vi "BST106-M10 Weighing Multicontroller Reporter.vi"() -> ()   [LabVIEW 2025]
uses:
  <vilib>/Utility/file.llb/Read Delimited Spreadsheet (string).vi
  Subprogramas/Variable global de carga.vi
  <vilib>/Utility/file.llb/Write Delimited Spreadsheet (string).vi
  <vilib>/Utility/error.llb/Error Cluster From Error Code.vi
  <vilib>/ErrorRing/Error Ring.xnode
  <vilib>/Plasmionique/MB Master/MB_Master_Serial/MB_Master_Serial.lvclass
panel:
  in  "Secret button":bool
  out "ReportXlsxPath":path=path "C:/Temp/Basculas Fabela MultiController/Documentos/Reporte.txt"
  out "CtrlClusterOld":T1(array[cluster])
  out "CtrlNumberOld":i32
  in  "ConfChange":bool caption="Lectura de controladores"
  out "PythonPath":path=path "C:/Temp/Insagro/Documentos/TXTaXLSX.exe"
  out "ReportPath":path=path "C:/Temp/Basculas Fabela MultiController/Documentos/Reporte.txt"
  out "ComNumberPath":path=path "C:/Temp/Basculas Fabela MultiController/Documentos/ComNumber.txt"
  out "ComConfigPath":path=path "C:/Temp/Basculas Fabela MultiController/Documentos/ComConfig.txt"
  out "TxtPath":path=path "C:/Temp/Basculas Fabela MultiController/Documentos/Recetas.txt"
  out "Tabs":enum32{"Home", "Main", "Setup"}(tab)=enum."Setup"
  in  "Controllers Load":T2(array[cluster])=[{"ControlerNum"="Controlador 1", "Recipe"="", "Status"=9868950}] caption="Controladores"
  in  "Carga total":bool
  out "Main Load":enum32{"No load", "Load"}(tab)
  out "Ring 2":u16(ring)
  in  "Read":bool caption="Lectura de controladores"
  out "Loading Text":string
  out "TABLA DE RECETAS":string[][](table)
  in  "SecretAnimationCtrl":i32=1 caption="Selección de animación secreta" min=1
  in  "Array CtrlCluster":T1(array[cluster])=[{"Control#"="Control 1", "Com"=""}]
  in  "CtrlNumber":i32=1 caption="Número de controladores" min=1
  in  "Boton Guardar Cambios":bool
  in  "Settings Nav Button":bool=TRUE
  in  "Recetas Nav Button":bool
  in  "Home Nav Button":bool
  # "Seleccione en cada pantalla la fórmula que desee servir"
  # "Peso Objetivo"
  # "Número de Fórmula"
  # "Peso Servido"
  # "Tolva 1"
  # "Tolva 2"
  # "Tolva 3"
  # "Tolva 4"
  # "Indicador Báscula Sirviendo"
  # "Botón Ajuste Manual"
  # "Indicador Falta Material"
  # "FORMULA SELECCIONADA"
  # "CONFIGURACION DE COMUNICACION"
  # "Seleccione los puertos de comunicación"
  # "Controladores"
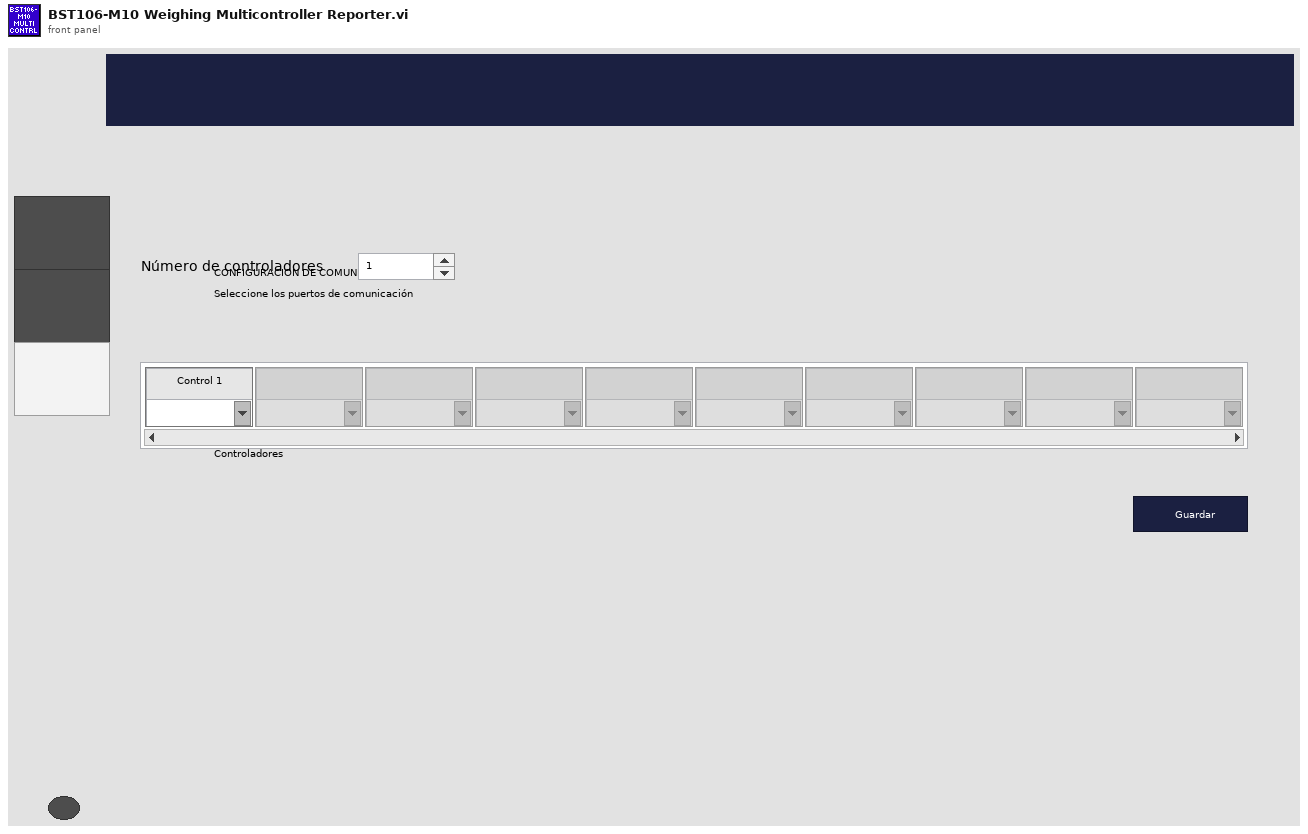
[diagram p1: front panel]
types:
  T1 = cluster{"Control#":string, "Com":refnum<visa-resource-name>}[]
  T2 = cluster{"ControlerNum":string, "Recipe":string, "Status":u32}[]
  T3 = enum8{"Enabled", "Disabled", "Disabled and Grayed Out"}
  T4 = cluster{"Control#":string, "Com":refnum<visa-resource-name>}
  T5 = cluster{"ControlerNum":string, "Recipe":string, "Status":u32}
  T6 = typedef "Control 2.ctl" = refnum<class "MB_Master_Serial.lvclass">[]
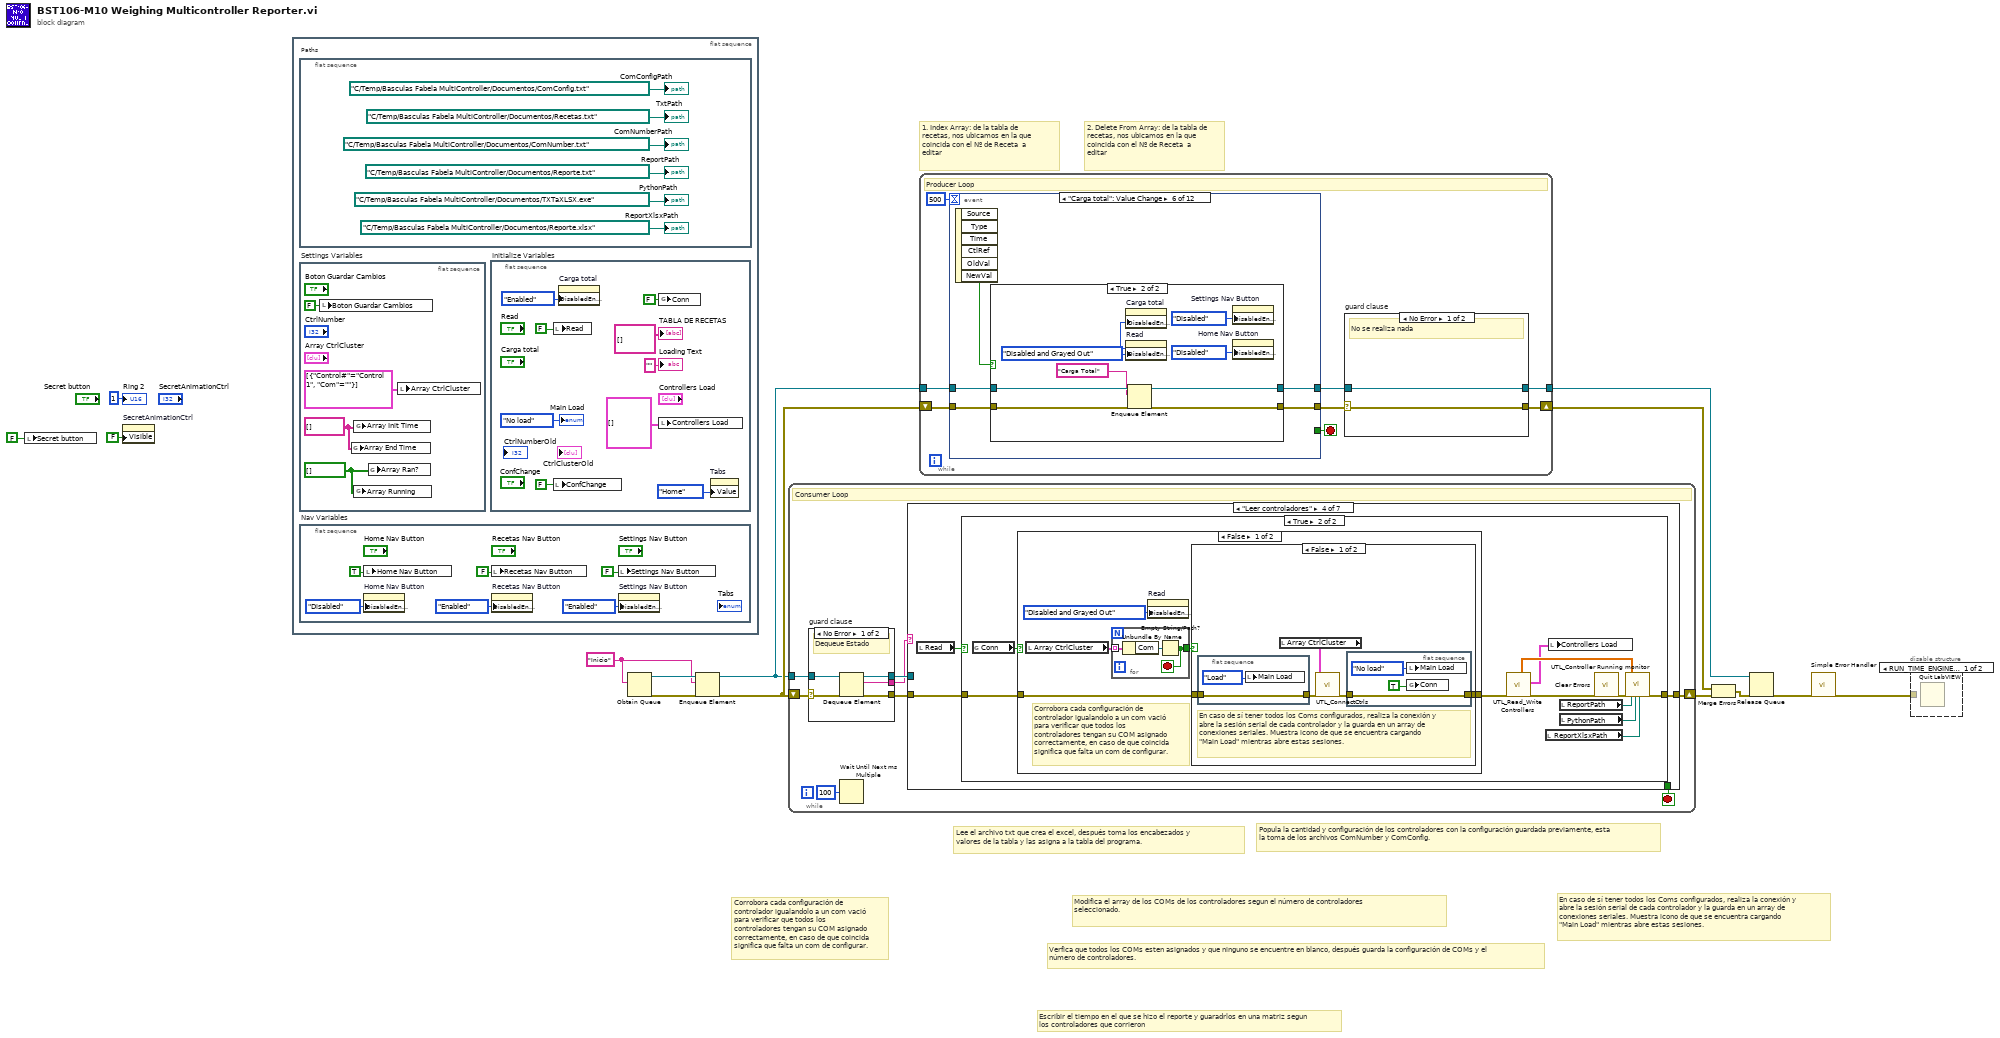
[diagram p0: block diagram]
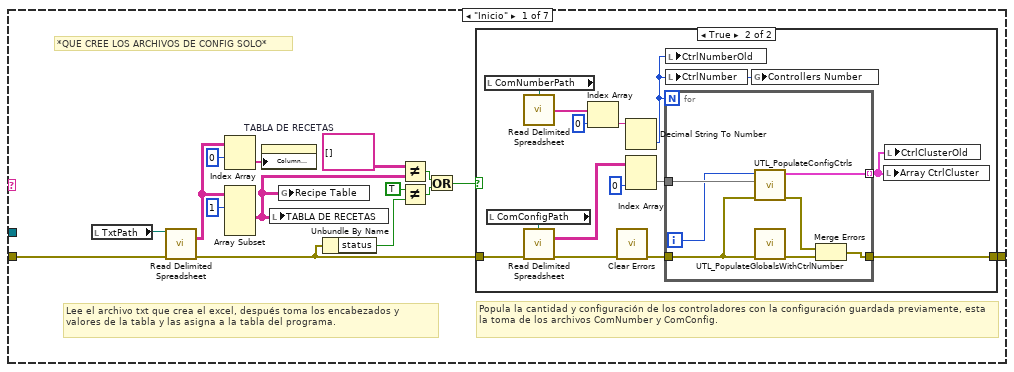
[diagram p2: hidden frame]
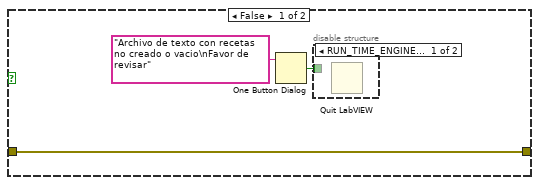
[diagram p3: hidden frame]
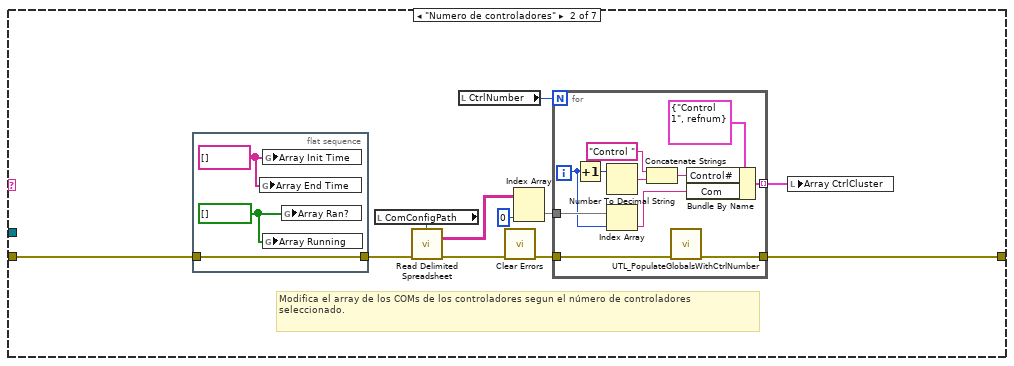
[diagram p5: hidden frame]
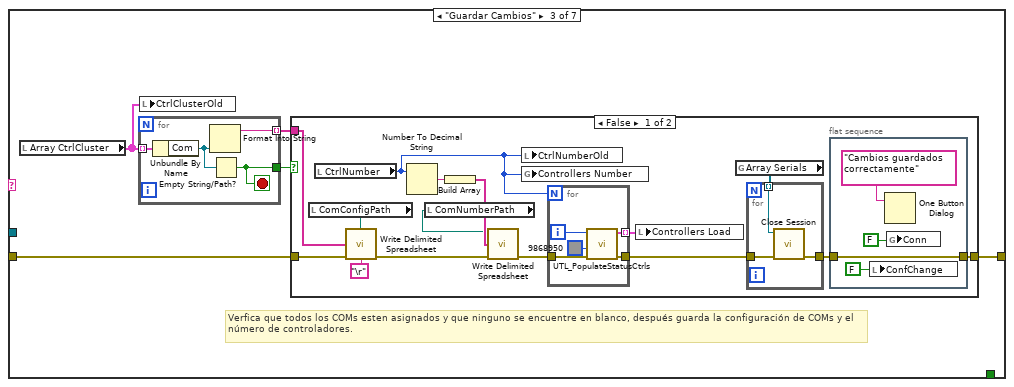
[diagram p6: hidden frame]
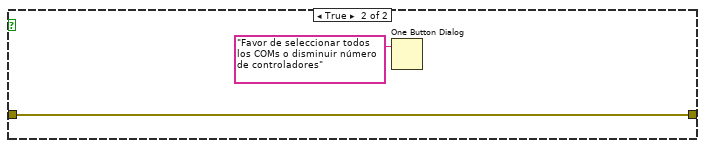
[diagram p7: hidden frame]
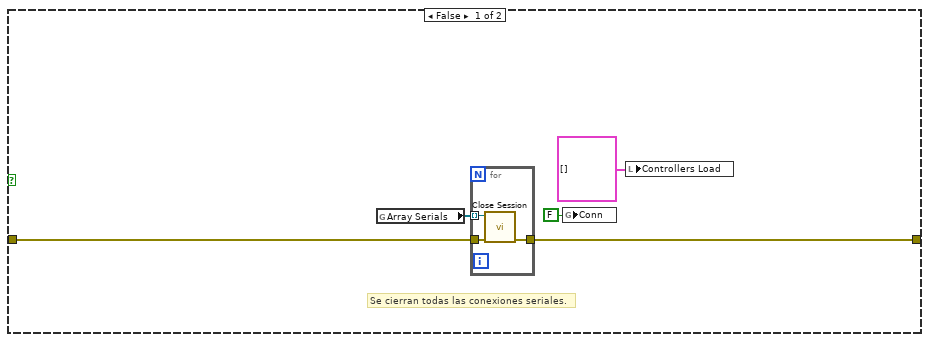
[diagram p8: hidden frame]
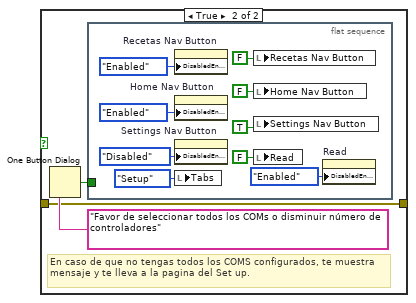
[diagram p9: hidden frame]
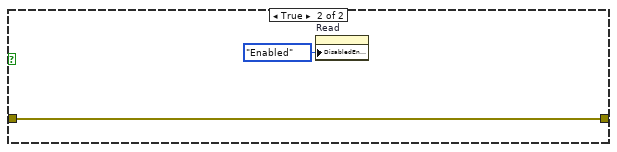
[diagram p10: hidden frame]
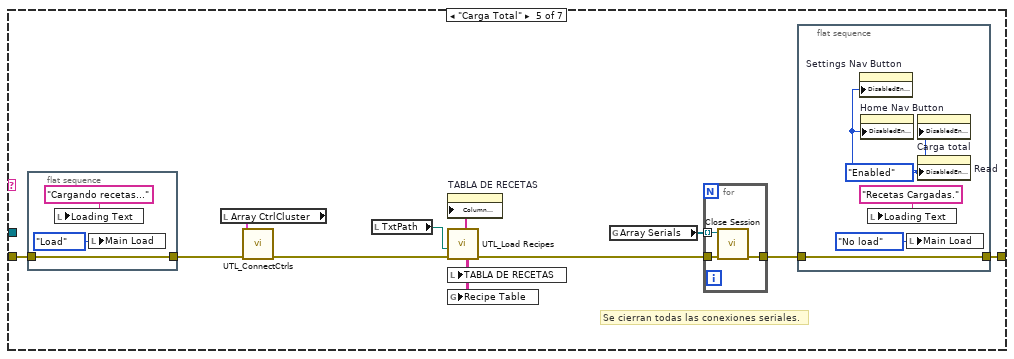
[diagram p11: hidden frame]
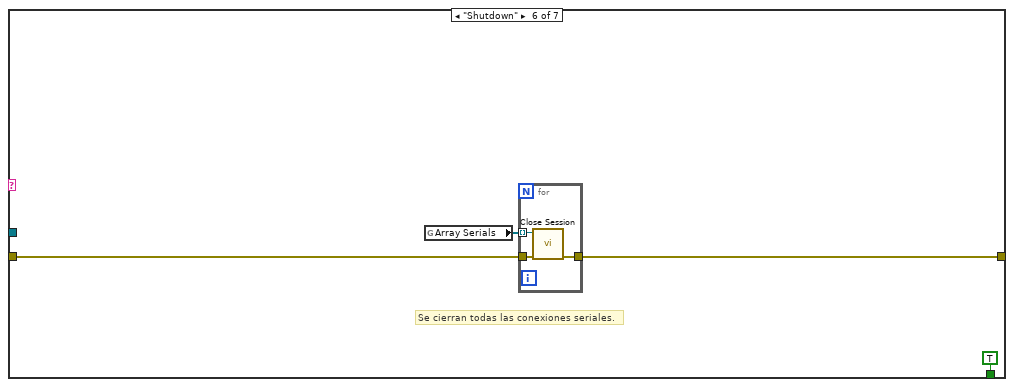
[diagram p12: hidden frame]
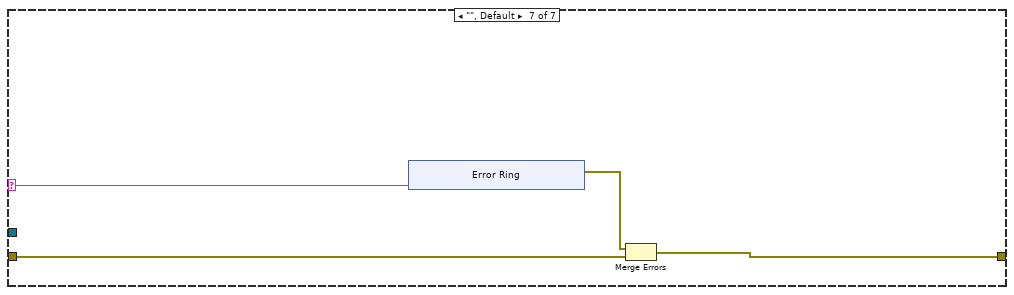
[diagram p13: hidden frame]
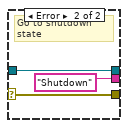
[diagram p14: hidden frame]
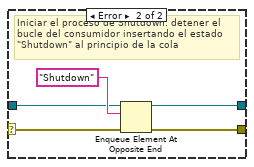
[diagram p15: hidden frame]
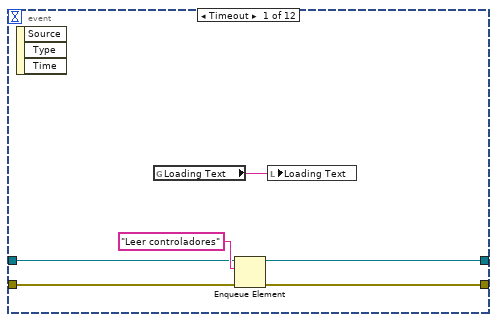
[diagram p16: hidden frame]
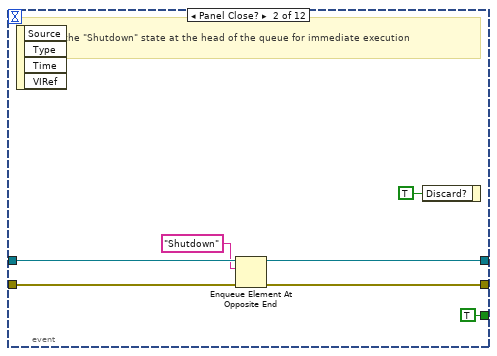
[diagram p17: hidden frame]
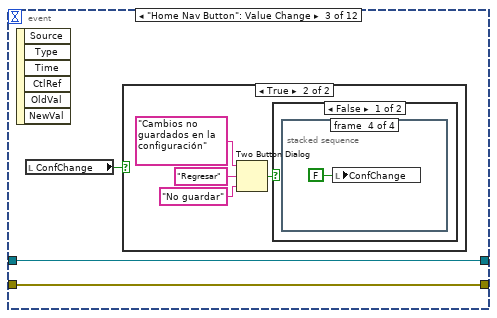
[diagram p18: hidden frame]
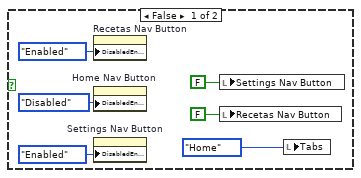
[diagram p19: hidden frame]
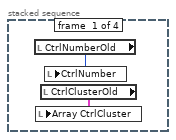
[diagram p20: hidden frame]
diagram:
  w5 = "Inicio"
  # "Escribir el tiempo en el que se hizo el reporte y guaradrlos en una matriz segun los controladores que corrieron"
  # "En caso de sí tener todos los Coms configurados, realiza la conexión y abre la sesión serial de cada controlador y la guarda en un array de conexiones seriales. Muestra icono de que se encuentra cargando \"Main Load\" mientras abre estas sesiones."
  # "Corrobora cada configuración de controlador igualandolo a un com vació para verificar que todos los controladores tengan su COM asignado correctamente, en caso de que coincida significa que falta un com de configurar."
  # "Verfica que todos los COMs esten asignados y que ninguno se encuentre en blanco, después guarda la configuración de COMs y el número de controladores."
  # "Modifica el array de los COMs de los controladores segun el número de controladores seleccionado."
  # "Popula la cantidad y configuración de los controladores con la configuración guardada previamente, esta la toma de los archivos ComNumber y ComConfig."
  # "Lee el archivo txt que crea el excel, después toma los encabezados y valores de la tabla y las asigna a la tabla del programa."
  # "2. Delete From Array: de la tabla de recetas, nos ubicamos en la que coincida con el Nº de Receta  a editar"
  # "1. Index Array: de la tabla de recetas, nos ubicamos en la que coincida con el Nº de Receta  a editar"
  n1 = local write "Secret button"(FALSE ("Secret button")) -> ()
  n2 = property on="SecretAnimationCtrl" class="DigNum (strict)"("Visible"=FALSE) -> ()  [unwired: 2 in, 2 out]
  n3 = flat-sequence {
    frame #0 {
      # "Initialize Variables"
      # "Nav Variables"
      # "Paths"
      # "Settings Variables"
      n4 = flat-sequence {
        frame #0 {
          "TxtPath" <- path "C:/Temp/Basculas Fabela MultiController/Documentos/Recetas.txt" ("name or relative path")
          "ComConfigPath" <- path "C:/Temp/Basculas Fabela MultiController/Documentos/ComConfig.txt" ("name or relative path")
          "ComNumberPath" <- path "C:/Temp/Basculas Fabela MultiController/Documentos/ComNumber.txt" ("name or relative path")
          "ReportPath" <- path "C:/Temp/Basculas Fabela MultiController/Documentos/Reporte.txt" ("name or relative path")
          "PythonPath" <- path "C:/Temp/Basculas Fabela MultiController/Documentos/TXTaXLSX.exe" ("name or relative path")
          "ReportXlsxPath" <- path "C:/Temp/Basculas Fabela MultiController/Documentos/Reporte.xlsx" ("name or relative path")
        }
      }
      n5 = flat-sequence {
        frame #0 {
          w38 = bool[] [] ("Array Ran?")
          w37 = string[] [] ("Array Init Time")
          n6 = local write "Boton Guardar Cambios"(FALSE ("Boton Iniciar programa")) -> ()
          n7 = global write "Variable global de carga.vi" "Array End Time"(w37) -> ()
          n8 = global write "Variable global de carga.vi" "Array Init Time"(w37) -> ()
          n9 = global write "Variable global de carga.vi" "Array Running"(w38) -> ()
          n10 = global write "Variable global de carga.vi" "Array Ran?"(w38) -> ()
          n11 = local write "Array CtrlCluster"(T1 [{"Control#"="Control 1", "Com"=""}] ("Array CtrlCluster")) -> ()
        }
      }
      n12 = flat-sequence {
        frame #0 {
          n13 = local write "Home Nav Button"(TRUE ("Home Nav Button")) -> ()
          n14 = property on="Home Nav Button" class="Bool (strict)"("DisabledEnum"=T3."Disabled" ("Disabled")) -> ()  [unwired: 2 in, 2 out]
          n15 = local write "Recetas Nav Button"(FALSE ("Recetas Nav Button")) -> ()
          n16 = property on="Recetas Nav Button" class="Bool (strict)"("DisabledEnum"=T3."Enabled" ("Disabled")) -> ()  [unwired: 2 in, 2 out]
          n17 = local write "Settings Nav Button"(FALSE ("Settings Nav Button")) -> ()
          n18 = property on="Settings Nav Button" class="Bool (strict)"("DisabledEnum"=T3."Enabled" ("Disabled")) -> ()  [unwired: 2 in, 2 out]
        }
      }
      n19 = flat-sequence {
        frame #0 {
          n20 = local write "Read"(FALSE ("Read")) -> ()
          n21 = local write "ConfChange"(FALSE ("ConfChange")) -> ()
          n22 = property on="Carga total" class="Bool (strict)"("DisabledEnum"=T3."Enabled" ("Disabled")) -> ()  [unwired: 2 in, 2 out]
          n23 = global write "Variable global de carga.vi" "Conn"(FALSE ("Conn")) -> ()
          n24 = local write "Controllers Load"(T2 [] ("Controllers Load")) -> ()
          n25 = property on="Tabs" class="TabCtl (strict)"("Value"=enum32{"Home", "Main", "Setup"}."Home" ("Tab Control")) -> ()  [unwired: 2 in, 2 out]
          "Main Load" <- enum32{"No load", "Load"}."No load" ("Load C1")
          "TABLA DE RECETAS" <- string[][] []
          "Loading Text" <- "" ("Variable de carga")
        }
      }
    }
  }
  n26 = Obtain Queue(element data type=w5) -> (queue out=w14:refnum<queue>, error out=w13:errorcluster)  [unwired: 4 in, 1 out]
  n27 = Enqueue Element(queue=w14, element=w5, error in (no error)=w13) -> (queue out=w8:refnum<queue>, error out=w9:errorcluster)  [unwired: 1 in, 1 out]
  n28 = while {
    shift-right: [w40] -> w11
    shift-left: w9 -> [w47]
    tunnel: w8 -> [w42]
    stop <- w43 stop-if-true
    # "Consumer Loop"
    n29 = case "guard clause" shown="No Error" w47 {
      selector: w47 -> [w247 w250]
      tunnel: [w246 "Shutdown"] -> w41
      tunnel: [w245 w248] -> w46
      tunnel: [w244 w250] -> w45
      tunnel: w42 -> [w243 w248]
      frame No Error {
        # "Dequeue Estado"
        n30 = Dequeue Element(queue=w243, error in (no error)=w247) -> (queue out=w245:refnum<queue>, element=w246:string, error out=w244:errorcluster)  [unwired: 1 in, 1 out]
      }
      frame Error {
        # "Go to shutdown state"
      }
    }
    n31 = Wait Until Next ms Multiple(millisecond multiple=u32 100) -> ()  [unwired: 1 out]
    n32 = case shown="\"Leer controladores\"" w41 {
      selector: w41 -> [_ _ _ _ _ _ w235]
      tunnel: w46 -> [_ _ _ _ _ _ _]
      tunnel: w45 -> [w53 w90 w113 w151 w214 w227 w234]
      tunnel: [_ _ _ _ _ TRUE _] -> w43
      tunnel: [w51 w87 w116 w150 w212 w226 w232] -> w40
      frame "Inicio" {
        # "*QUE CREE LOS ARCHIVOS DE CONFIG SOLO*"
        # "Popula la cantidad y configuración de los controladores con la configuración guardada previamente, esta la toma de los archivos ComNumber y ComConfig."
        # "Lee el archivo txt que crea el excel, después toma los encabezados y valores de la tabla y las asigna a la tabla del programa."
        n33 = local read "TxtPath"() -> (w56:path)
        n34 = call-poly <vilib>:"Read Delimited Spreadsheet.vi"("file path (dialog if empty)"=w56, "error in (no error)"=w53) -> ("all rows"=w61:string[][], "error out"=w52:errorcluster)  [unwired: 8 in, 4 out]
        n35 = Index Array(array=w61, index (row)=0) -> (element=w62:string[])  [unwired: 1 in]
        n36 = Array Subset(array=w61, index (row)=1 ("index")) -> (w50:string[][])  [unwired: 3 in]
        n37 = property on="TABLA DE RECETAS" class="Tbl (strict)"("Column Headers[]"=w62) -> ()  [unwired: 2 in, 2 out]
        n38 = local write "TABLA DE RECETAS"(w50) -> ()
        n39 = global write "Variable global de carga.vi" "Recipe Table"(w50) -> ()
        n40 = Unbundle By Name(w52) -> ("status"=w59:bool)
        n41 = Not Equal?(x=string[][] [], y=w50) -> (x != y?=w58:bool)
        n42 = Not Equal?(x=TRUE, y=w59) -> (x != y?=w60:bool)
        n43 = Or(x=w58, y=w60) -> (x .or. y?=w57:bool)
        n44 = case shown="True" w57 {
          tunnel: w52 -> [w63 w75]
          tunnel: [w63 w68] -> w51
          frame False {
            n45 = One Button Dialog(message="Archivo de texto con recetas no creado o vacio\nFavor de revisar") -> (true=w64:bool)  [unwired: 1 in]
            n46 = disable-structure shown="RUN_TIME_ENGINE==True" {
              disable-tunnel: w64 -> [_ _]
              frame condition #0 {
                n47 = Quit LabVIEW() -> ()  [unwired: 1 in]
              }
              frame condition #1 (active) {
              }
            }
          }
          frame True {
            n48 = local read "ComNumberPath"() -> (w74:path)
            n49 = local read "ComConfigPath"() -> (w76:path)
            n50 = call-poly <vilib>:"Read Delimited Spreadsheet.vi"("file path (dialog if empty)"=w74) -> ("first row"=w73:string[])  [unwired: 9 in, 5 out]
            n51 = call-poly <vilib>:"Read Delimited Spreadsheet.vi"("file path (dialog if empty)"=w76, "error in (no error)"=w75) -> ("all rows"=w79:string[][], "error out"=w77:errorcluster)  [unwired: 8 in, 4 out]
            n52 = Index Array(array=w73, index=0 ("disabled index (col)")) -> (element=w72:string)
            n53 = call <vilib>:"Clear Errors.vi"("error in (no error)"=w77) -> ("error out"=w69:errorcluster)  [unwired: 5 in, 1 out]
            n54 = Decimal String To Number(string=w72) -> (number=w66:i32)  [unwired: 2 in, 1 out]
            n55 = Index Array(array=w79, index (col)=0 ("disabled index (col)")) -> (element=w70:string[])  [unwired: 1 in]
            n56 = for {
              N: w66 -> [_]
              tunnel: w70 -> [w86]
              tunnel: w69 -> [w82]
              tunnel: [w83] -> w68
              tunnel: [w85] -> w67 mode=indexing
              i -> [w81]
              n57 = call "UTL_PopulateConfigCtrls.vi"("error in (no error)"=w82, "ComConfig"=w86, "ComNum"=w81) -> ("error out"=w80:errorcluster, "Array Cluster"=w85:T4)  [unwired: 7 in]
              n58 = call "UTL_PopulateGlobalsWithCtrlNumber.vi"("error in (no error)"=w82) -> ("error out"=w84:errorcluster)  [unwired: 10 in]
              n59 = Merge Errors(w80, w84) -> (w83:errorcluster)
            }
            n60 = local write "CtrlNumberOld"(w66) -> ()
            n61 = local write "CtrlNumber"(w66) -> ()
            n62 = global write "Variable global de carga.vi" "Controllers Number"(w66) -> ()
            n63 = local write "Array CtrlCluster"(w67) -> ()
            n64 = local write "CtrlClusterOld"(w67) -> ()
          }
        }
      }
      frame "Numero de controladores" {
        # "Modifica el array de los COMs de los controladores segun el número de controladores seleccionado."
        n65 = flat-sequence {
          tunnel: w90 -> [w98]
          tunnel: [w98] -> w89
          frame #0 {
            w100 = bool[] [] ("Array Ran?")
            w99 = string[] [] ("Array Init Time")
            n66 = global write "Variable global de carga.vi" "Array End Time"(w99) -> ()
            n67 = global write "Variable global de carga.vi" "Array Init Time"(w99) -> ()
            n68 = global write "Variable global de carga.vi" "Array Running"(w100) -> ()
            n69 = global write "Variable global de carga.vi" "Array Ran?"(w100) -> ()
          }
        }
        n70 = local read "ComConfigPath"() -> (w95:path)
        n71 = call-poly <vilib>:"Read Delimited Spreadsheet.vi"("file path (dialog if empty)"=w95, "error in (no error)"=w89) -> ("all rows"=w97:string[][], "error out"=w96:errorcluster)  [unwired: 8 in, 4 out]
        n72 = local read "CtrlNumber"() -> (w91:i32)
        n73 = call <vilib>:"Clear Errors.vi"("error in (no error)"=w96) -> ("error out"=w88:errorcluster)  [unwired: 5 in, 1 out]
        n74 = Index Array(array=w97, index (col)=0 ("disabled index (col)")) -> (element=w94:string[])  [unwired: 1 in]
        n75 = for {
          N: w91 -> [_]
          tunnel: w94 -> [w105]
          tunnel: [w106] -> w93 mode=indexing
          tunnel: w88 -> [w102]
          tunnel: [w101] -> w87
          i -> [w104]
          n76 = Increment(x=w104) -> (x+1=w107:i32)
          n77 = Number To Decimal String(number=w107) -> (decimal integer string=w111:string)  [unwired: 1 in]
          n78 = Index Array(array=w105, index=w104) -> (element=w103:string)
          n79 = Concatenate Strings("Control " ("Control#"), w111) -> (w110:string)
          n80 = call "UTL_PopulateGlobalsWithCtrlNumber.vi"("error in (no error)"=w102) -> ("error out"=w101:errorcluster)  [unwired: 10 in]
          n81 = Bundle By Name(cluster=T4 {"Control#"="Control 1", "Com"=""} ("CtrlClust"), "Control#"=w110, "Com"=w103) -> (w106:T4)
        }
        n82 = local write "Array CtrlCluster"(w93) -> ()
      }
      frame "Guardar Cambios" {
        # "Verfica que todos los COMs esten asignados y que ninguno se encuentre en blanco, después guarda la configuración de COMs y el número de controladores."
        n83 = local read "Array CtrlCluster"() -> (w112:T1)
        n84 = for {
          tunnel: [w146] -> w114
          tunnel: [w149] -> w115 mode=indexing
          tunnel: w112 -> [w148] mode=indexing
          stop <- w146 stop-if-true
          n85 = Unbundle By Name(w148) -> ("Com"=w147:refnum<visa-resource-name>)
          n86 = Format Into String(w147) -> (resulting string=w149:string)  [unwired: 3 in, 1 out]
          n87 = Empty String/Path?(string/path=w147) -> (empty?=w146:bool)
        }
        n88 = local write "CtrlClusterOld"(w112) -> ()
        n89 = case shown="False" w114 {
          tunnel: w115 -> [w130 _]
          tunnel: [w126 w144] -> w116
          tunnel: w113 -> [w129 w144]
          frame False {
            n90 = local read "ComConfigPath"() -> (w128:path)
            n91 = local read "CtrlNumber"() -> (w117:i32)
            n92 = call-poly <vilib>:"Write Delimited Spreadsheet.vi"("file path (dialog if empty)"=w128, "1D data"=w130, "error in (no error)"=w129, "delimiter (\\t)"="\r") -> ("error out"=w122:errorcluster)  [unwired: 10 in, 1 out]
            n93 = Number To Decimal String(number=w117) -> (decimal integer string=w124:string)  [unwired: 1 in]
            n94 = local read "ComNumberPath"() -> (w121:path)
            n95 = Build Array(w124) -> (w123:string[])
            n96 = call-poly <vilib>:"Write Delimited Spreadsheet.vi"("file path (dialog if empty)"=w121, "1D data"=w123, "error in (no error)"=w122) -> ("error out"=w120:errorcluster)  [unwired: 11 in, 1 out]
            n97 = local write "CtrlNumberOld"(w117) -> ()
            n98 = global write "Variable global de carga.vi" "Controllers Number"(w117) -> ()
            n99 = for {
              N: w117 -> [_]
              tunnel: w120 -> [w136]
              tunnel: [w135] -> w119
              tunnel: [w132] -> w118 mode=indexing
              i -> [w133]
              n100 = call "UTL_PopulateStatusCtrls.vi"("error in (no error)"=w136, "Status"=u32 9868950, "ComNum"=w133) -> ("error out"=w135:errorcluster, "output cluster"=w132:T5)  [unwired: 7 in]
            }
            n101 = local write "Controllers Load"(w118) -> ()
            n102 = global read "Variable global de carga.vi" "Array Serials"() -> (w125:T6)
            n103 = for {
              tunnel: [w143] -> w127
              tunnel: w119 -> [w142]
              tunnel: w125 -> [w141] mode=indexing
              n104 = call-dynamic "Close Session.vi"("error in (no error)"=w142, "MB_Serial session"=w141) -> ("error out"=w143:errorcluster)  [unwired: 9 in]
            }
            n105 = flat-sequence {
              tunnel: w127 -> [w140]
              tunnel: [w140] -> w126
              frame #0 {
                n106 = local write "ConfChange"(FALSE ("ConfChange")) -> ()
                n107 = One Button Dialog(message="Cambios guardados correctamente") -> ()  [unwired: 1 in, 1 out]
                n108 = global write "Variable global de carga.vi" "Conn"(FALSE ("Conn")) -> ()
              }
            }
          }
          frame True {
            n109 = One Button Dialog(message="Favor de seleccionar todos los COMs o disminuir número de controladores") -> ()  [unwired: 1 in, 1 out]
          }
        }
      }
      frame "Leer controladores" {
        n110 = local read "Read"() -> (w152:bool)
        n111 = case shown="True" w152 {
          tunnel: [w155 w171] -> w150
          tunnel: w151 -> [w156 w165]
          frame False {
            # "Se cierran todas las conexiones seriales."
            n112 = global read "Variable global de carga.vi" "Array Serials"() -> (w157:T6)
            n113 = for {
              tunnel: [w160] -> w155
              tunnel: w156 -> [w159]
              tunnel: w157 -> [w158] mode=indexing
              n114 = call-dynamic "Close Session.vi"("error in (no error)"=w159, "MB_Serial session"=w158) -> ("error out"=w160:errorcluster)  [unwired: 9 in]
            }
            n115 = global write "Variable global de carga.vi" "Conn"(FALSE ("Conn")) -> ()
            n116 = local write "Controllers Load"(T2 [] ("Controllers Load")) -> ()
          }
          frame True {
            n117 = global read "Variable global de carga.vi" "Conn"() -> (w167:bool)
            n118 = case shown="False" w167 {
              tunnel: [w176 w203] -> w166
              tunnel: w165 -> [w173 w203]
              frame False {
                # "Corrobora cada configuración de controlador igualandolo a un com vació para verificar que todos los controladores tengan su COM asignado correctamente, en caso de que coincida significa que falta un com de configurar."
                n119 = local read "Array CtrlCluster"() -> (w174:T1)
                n120 = for {
                  tunnel: [w177] -> w175
                  tunnel: w174 -> [w179] mode=indexing
                  stop <- w177 stop-if-true
                  n121 = Unbundle By Name(w179) -> ("Com"=w178:refnum<visa-resource-name>)
                  n122 = Empty String/Path?(string/path=w178) -> (empty?=w177:bool)
                }
                n123 = property on="Read" class="Bool (strict)"("DisabledEnum"=T3."Disabled and Grayed Out" ("Disabled")) -> ()  [unwired: 2 in, 2 out]
                n124 = case shown="False" w175 {
                  tunnel: [w184 w190] -> w176
                  tunnel: w173 -> [w180 w190]
                  frame False {
                    # "En caso de sí tener todos los Coms configurados, realiza la conexión y abre la sesión serial de cada controlador y la guarda en un array de conexiones seriales. Muestra icono de que se encuentra cargando \"Main Load\" mientras abre estas sesiones."
                    n125 = flat-sequence {
                      tunnel: [w188] -> w181
                      tunnel: w180 -> [w188]
                      frame #0 {
                        n126 = local write "Main Load"(enum32{"No load", "Load"}."Load" ("Load C1")) -> ()
                      }
                    }
                    n127 = local read "Array CtrlCluster"() -> (w182:T1)
                    n128 = call "UTL_ConnectCtrls.vi"("error in (no error)"=w181, "Array CtrlCluster"=w182) -> ("error out"=w183:errorcluster)  [unwired: 9 in]
                    n129 = flat-sequence {
                      tunnel: w183 -> [w186]
                      tunnel: [w186] -> w184
                      frame #0 {
                        n130 = local write "Main Load"(enum32{"No load", "Load"}."No load" ("Load C1")) -> ()
                        n131 = global write "Variable global de carga.vi" "Conn"(TRUE ("Conn")) -> ()
                      }
                    }
                  }
                  frame True {
                    # "En caso de que no tengas todos los COMS configurados, te muestra mensaje y te lleva a la pagina del Set up."
                    n132 = One Button Dialog(message="Favor de seleccionar todos los COMs o disminuir número de controladores") -> (true=w191:bool)  [unwired: 1 in]
                    n133 = flat-sequence {
                      tunnel: w191 -> [_]
                      frame #0 {
                        n134 = property on="Recetas Nav Button" class="Bool (strict)"("DisabledEnum"=T3."Enabled" ("Disabled")) -> ()  [unwired: 2 in, 2 out]
                        n135 = property on="Home Nav Button" class="Bool (strict)"("DisabledEnum"=T3."Enabled" ("Disabled")) -> ()  [unwired: 2 in, 2 out]
                        n136 = property on="Settings Nav Button" class="Bool (strict)"("DisabledEnum"=T3."Disabled" ("Disabled")) -> ()  [unwired: 2 in, 2 out]
                        n137 = local write "Tabs"(enum32{"Home", "Main", "Setup"}."Setup" ("Pagina programa")) -> ()
                        n138 = local write "Recetas Nav Button"(FALSE ("Recetas Nav Button")) -> ()
                        n139 = local write "Home Nav Button"(FALSE ("Settings Nav Button")) -> ()
                        n140 = local write "Settings Nav Button"(TRUE ("Settings Nav Button")) -> ()
                        n141 = local write "Read"(FALSE ("Read")) -> ()
                        n142 = property on="Read" class="Bool (strict)"("DisabledEnum"=T3."Enabled" ("Disabled")) -> ()  [unwired: 2 in, 2 out]
                      }
                    }
                  }
                }
              }
              frame True {
                n143 = property on="Read" class="Bool (strict)"("DisabledEnum"=T3."Enabled" ("Disabled")) -> ()  [unwired: 2 in, 2 out]
              }
            }
            n144 = call "UTL_Read_Write Controllers.vi"("error in"=w166) -> ("error out"=w170:errorcluster, "StatusCtrl"=w168:T2, "Results"=w169:dbl[][][])  [unwired: 8 in]
            n145 = local read "ReportXlsxPath"() -> (w161:path)
            n146 = local write "Controllers Load"(w168) -> ()
            n147 = local read "ReportPath"() -> (w163:path)
            n148 = local read "PythonPath"() -> (w162:path)
            n149 = call <vilib>:"Clear Errors.vi"("error in (no error)"=w170) -> ("error out"=w164:errorcluster)  [unwired: 5 in, 1 out]
            n150 = call "UTL_Controller Running monitor.vi"("Error In"=w164, "Data"=w169, "ReportPath"=w163, "PyPath"=w162, "ReportXlsxPath"=w161) -> ("Error Out"=w171:errorcluster)  [unwired: 14 in]
          }
        }
      }
      frame "Carga Total" {
        # "Se cierran todas las conexiones seriales."
        n151 = flat-sequence {
          tunnel: w214 -> [w223]
          tunnel: [w223] -> w208
          frame #0 {
            n152 = local write "Loading Text"("Cargando recetas..." ("Carga texto")) -> ()
            n153 = local write "Main Load"(enum32{"No load", "Load"}."Load" ("Load C1")) -> ()
          }
        }
        n154 = local read "Array CtrlCluster"() -> (w209:T1)
        n155 = call "UTL_ConnectCtrls.vi"("error in (no error)"=w208, "Array CtrlCluster"=w209) -> ("error out"=w207:errorcluster)  [unwired: 9 in]
        n156 = local read "TxtPath"() -> (w213:path)
        n157 = call "UTL_Load Recipes.vi"("Error in"=w207, "Txt Path"=w213) -> ("Error out"=w205:errorcluster, "Headers"=w210:string[], "Sorted 2D table array"=w211:string[][])  [unwired: 7 in]
        n158 = property on="TABLA DE RECETAS" class="Tbl (strict)"("Column Headers[]"=w210) -> ()  [unwired: 2 in, 2 out]
        n159 = local write "TABLA DE RECETAS"(w211) -> ()
        n160 = global write "Variable global de carga.vi" "Recipe Table"(w211) -> ()
        n161 = global read "Variable global de carga.vi" "Array Serials"() -> (w206:T6)
        n162 = for {
          tunnel: [w217] -> w204
          tunnel: w205 -> [w216]
          tunnel: w206 -> [w215] mode=indexing
          n163 = call-dynamic "Close Session.vi"("error in (no error)"=w216, "MB_Serial session"=w215) -> ("error out"=w217:errorcluster)  [unwired: 9 in]
        }
        n164 = flat-sequence {
          tunnel: w204 -> [w220]
          tunnel: [w220] -> w212
          frame #0 {
            w218 = T3."Enabled" ("Disabled")
            n165 = property on="Settings Nav Button" class="Bool (strict)"("DisabledEnum"=w218) -> ()  [unwired: 2 in, 2 out]
            n166 = property on="Home Nav Button" class="Bool (strict)"("DisabledEnum"=w218) -> ()  [unwired: 2 in, 2 out]
            n167 = local write "Loading Text"("Recetas Cargadas." ("Carga texto")) -> ()
            n168 = local write "Main Load"(enum32{"No load", "Load"}."No load" ("Load C1")) -> ()
            n169 = property on="Carga total" class="Bool (strict)"("DisabledEnum"=w218) -> ()  [unwired: 2 in, 2 out]
            n170 = property on="Read" class="Bool (strict)"("DisabledEnum"=w218) -> ()  [unwired: 2 in, 2 out]
          }
        }
      }
      frame "Shutdown" {
        # "Se cierran todas las conexiones seriales."
        # "Stop the Consumer Loop, and signal the Producer Loop to also stop by activating the front-panel \"Stop\" button; use the \"signaling\" version to trigger the event structure"
        n171 = global read "Variable global de carga.vi" "Array Serials"() -> (w225:T6)
        n172 = for {
          tunnel: [w231] -> w226
          tunnel: w227 -> [w230]
          tunnel: w225 -> [w229] mode=indexing
          n173 = call-dynamic "Close Session.vi"("error in (no error)"=w230, "MB_Serial session"=w229) -> ("error out"=w231:errorcluster)  [unwired: 9 in]
        }
      }
      frame "", Default {
        # "Handle unknown states"
        n174 = xnode "Error Ring"("parameter 0"=w235) -> ("error out"=w233:errorcluster)
        n175 = Merge Errors(w233, w234) -> (w232:errorcluster)
      }
    }
  }
  n176 = while {
    shift-right: [w253] -> w7
    shift-left: w9 -> [w257]
    tunnel: w8 -> [w256]
    tunnel: [w254] -> w6
    stop <- w252 stop-if-true
    # "Producer Loop"
    n177 = event shown="[5] \"Carga total\": Value Change" {
      selector: _ -> [_ _ _ _ _ _ _ _ _ _ _ _]
      dyn-events: _ -> [_ _ _ _ _ _ _ _ _ _ _ _]
      timeout: 500 -> [_ _ _ _ _ _ _ _ _ _ _ _]
      tunnel: [w268 w275 w280 w306 w335 w339 w356 w364 w371 _ _ w387] -> w258
      tunnel: w257 -> [w269 w276 w280 w306 w335 w340 w357 w364 w371 _ _ w388]
      tunnel: w256 -> [w266 w278 w281 w305 w334 w341 w359 w365 w370 _ _ w389]
      tunnel: [_ TRUE _ _ _ _ _ _ _ _ _ _] -> w252
      tunnel: [w267 w273 w281 w305 w334 w338 w355 w365 w370 _ _ w386] -> w255
      event Timeout {
        n178 = event-data() -> ()  [unwired: 1 in, 3 out]
        n179 = global read "Variable global de carga.vi" "Loading Text"() -> (w271:string)
        n180 = Enqueue Element(queue=w266, element="Leer controladores", error in (no error)=w269) -> (queue out=w267:refnum<queue>, error out=w268:errorcluster)  [unwired: 1 in, 1 out]
        n181 = local write "Loading Text"(w271) -> ()
      }
      event Panel Close? {
        # "Enqueue the \"Shutdown\" state at the head of the queue for immediate execution"
        n182 = event-data() -> ()  [unwired: 1 in, 4 out]
        n183 = Enqueue Element At Opposite End(queue=w278, element="Shutdown", error in (no error)=w276) -> (queue out=w273:refnum<queue>, error out=w275:errorcluster)  [unwired: 1 in, 1 out]
        n184 = event-data("Discard?"=TRUE) -> ()  [unwired: 1 in, 1 out]
      }
      event "Home Nav Button": Value Change {
        n185 = event-data() -> ()  [unwired: 1 in, 6 out]
        n186 = local read "ConfChange"() -> (w279:bool)
        n187 = case shown="True" w279 {
          frame False {
            n188 = property on="Recetas Nav Button" class="Bool (strict)"("DisabledEnum"=T3."Enabled" ("Disabled")) -> ()  [unwired: 2 in, 2 out]
            n189 = property on="Home Nav Button" class="Bool (strict)"("DisabledEnum"=T3."Disabled" ("Disabled")) -> ()  [unwired: 2 in, 2 out]
            n190 = property on="Settings Nav Button" class="Bool (strict)"("DisabledEnum"=T3."Enabled" ("Disabled")) -> ()  [unwired: 2 in, 2 out]
            n191 = local write "Settings Nav Button"(FALSE ("Settings Nav Button")) -> ()
            n192 = local write "Recetas Nav Button"(FALSE ("Recetas Nav Button")) -> ()
            n193 = local write "Tabs"(enum32{"Home", "Main", "Setup"}."Home" ("Pagina programa")) -> ()
          }
          frame True {
            n194 = Two Button Dialog(message="Cambios no guardados en la configuración", 1:"No guardar" ("F button name (\"Cancel\")"), 2:"Regresar" ("T button name (\"OK\")")) -> (T button?=w288:bool)
            n195 = case shown="False" w288 {
              frame False {
                n196 = stacked-sequence {
                  frame #0 {
                    n197 = local read "CtrlNumberOld"() -> (w292:i32)
                    n198 = local read "CtrlClusterOld"() -> (w293:T1)
                    n199 = local write "Array CtrlCluster"(w293) -> ()
                    n200 = local write "CtrlNumber"(w292) -> ()
                  }
                  frame #1 {
                    w295 = T3."Enabled" ("Disabled")
                    n201 = property on="Settings Nav Button" class="Bool (strict)"("DisabledEnum"=w295) -> ()  [unwired: 2 in, 2 out]
                    n202 = property on="Recetas Nav Button" class="Bool (strict)"("DisabledEnum"=w295) -> ()  [unwired: 2 in, 2 out]
                    n203 = property on="Home Nav Button" class="Bool (strict)"("DisabledEnum"=T3."Disabled" ("Disabled")) -> ()  [unwired: 2 in, 2 out]
                  }
                  frame #2 {
                    n204 = local write "Settings Nav Button"(FALSE ("Settings Nav Button")) -> ()
                    n205 = local write "Recetas Nav Button"(FALSE ("Recetas Nav Button")) -> ()
                    n206 = local write "Tabs"(enum32{"Home", "Main", "Setup"}."Home" ("Pagina programa")) -> ()
                  }
                  frame #3 {
                    n207 = local write "ConfChange"(FALSE ("ConfChange")) -> ()
                  }
                }
              }
              frame True {
                n208 = local write "Recetas Nav Button"(FALSE ("Recetas Nav Button")) -> ()
                n209 = local write "Home Nav Button"(FALSE ("Settings Nav Button")) -> ()
                n210 = local write "Settings Nav Button"(TRUE ("Settings Nav Button")) -> ()
                n211 = local write "Tabs"(enum32{"Home", "Main", "Setup"}."Setup" ("Pagina programa")) -> ()
              }
            }
          }
        }
      }
      event "Recetas Nav Button": Value Change {
        n212 = event-data() -> ()  [unwired: 1 in, 6 out]
        n213 = local read "ConfChange"() -> (w304:bool)
        n214 = case shown="True" w304 {
          frame False {
            n215 = property on="Recetas Nav Button" class="Bool (strict)"("DisabledEnum"=T3."Disabled" ("Disabled")) -> ()  [unwired: 2 in, 2 out]
            n216 = property on="Home Nav Button" class="Bool (strict)"("DisabledEnum"=T3."Enabled" ("Disabled")) -> ()  [unwired: 2 in, 2 out]
            n217 = property on="Settings Nav Button" class="Bool (strict)"("DisabledEnum"=T3."Enabled" ("Disabled")) -> ()  [unwired: 2 in, 2 out]
            n218 = local write "Home Nav Button"(FALSE ("Recetas Nav Button")) -> ()
            n219 = local write "Settings Nav Button"(FALSE ("Settings Nav Button")) -> ()
            n220 = local write "Tabs"(enum32{"Home", "Main", "Setup"}."Main" ("Pagina programa")) -> ()
          }
          frame True {
            n221 = Two Button Dialog(message="Cambios no guardados en la configuración", 1:"No guardar" ("F button name (\"Cancel\")"), 2:"Regresar" ("T button name (\"OK\")")) -> (T button?=w316:bool)
            n222 = case shown="False" w316 {
              frame False {
                n223 = stacked-sequence {
                  frame #0 {
                    n224 = local read "CtrlNumberOld"() -> (w317:i32)
                    n225 = local read "CtrlClusterOld"() -> (w318:T1)
                    n226 = local write "Array CtrlCluster"(w318) -> ()
                    n227 = local write "CtrlNumber"(w317) -> ()
                  }
                  frame #1 {
                    w320 = T3."Enabled" ("Disabled")
                    n228 = property on="Recetas Nav Button" class="Bool (strict)"("DisabledEnum"=T3."Disabled" ("Disabled")) -> ()  [unwired: 2 in, 2 out]
                    n229 = property on="Home Nav Button" class="Bool (strict)"("DisabledEnum"=w320) -> ()  [unwired: 2 in, 2 out]
                    n230 = property on="Settings Nav Button" class="Bool (strict)"("DisabledEnum"=w320) -> ()  [unwired: 2 in, 2 out]
                  }
                  frame #2 {
                    n231 = local write "Home Nav Button"(FALSE ("Recetas Nav Button")) -> ()
                    n232 = local write "Settings Nav Button"(FALSE ("Settings Nav Button")) -> ()
                    n233 = local write "Tabs"(enum32{"Home", "Main", "Setup"}."Main" ("Pagina programa")) -> ()
                  }
                  frame #3 {
                    n234 = local write "ConfChange"(FALSE ("ConfChange")) -> ()
                  }
                }
              }
              frame True {
                n235 = local write "Recetas Nav Button"(FALSE ("Recetas Nav Button")) -> ()
                n236 = local write "Home Nav Button"(FALSE ("Settings Nav Button")) -> ()
                n237 = local write "Settings Nav Button"(TRUE ("Settings Nav Button")) -> ()
                n238 = local write "Tabs"(enum32{"Home", "Main", "Setup"}."Setup" ("Pagina programa")) -> ()
              }
            }
          }
        }
      }
      event "Settings Nav Button": Value Change {
        n239 = event-data() -> ()  [unwired: 1 in, 6 out]
        n240 = property on="Recetas Nav Button" class="Bool (strict)"("DisabledEnum"=T3."Enabled" ("Disabled")) -> ()  [unwired: 2 in, 2 out]
        n241 = property on="Home Nav Button" class="Bool (strict)"("DisabledEnum"=T3."Enabled" ("Disabled")) -> ()  [unwired: 2 in, 2 out]
        n242 = property on="Settings Nav Button" class="Bool (strict)"("DisabledEnum"=T3."Disabled" ("Disabled")) -> ()  [unwired: 2 in, 2 out]
        n243 = local write "Home Nav Button"(FALSE ("Recetas Nav Button")) -> ()
        n244 = local write "Recetas Nav Button"(FALSE ("Recetas Nav Button")) -> ()
        n245 = local write "Tabs"(enum32{"Home", "Main", "Setup"}."Setup" ("Pagina programa")) -> ()
      }
      event "Carga total": Value Change {
        n246 = event-data() -> ("NewVal"=w337:bool)  [unwired: 1 in, 5 out]
        n247 = case shown="True" w337 {
          tunnel: w341 -> [w343 w351]
          tunnel: w340 -> [w342 w349]
          tunnel: [w342 w348] -> w339
          tunnel: [w343 w347] -> w338
          frame False {
          }
          frame True {
            w346 = T3."Disabled and Grayed Out" ("Disabled")
            n248 = property on="Carga total" class="Bool (strict)"("DisabledEnum"=w346) -> ()  [unwired: 2 in, 2 out]
            n249 = property on="Read" class="Bool (strict)"("DisabledEnum"=w346) -> ()  [unwired: 2 in, 2 out]
            n250 = Enqueue Element(queue=w351, element="Carga Total", error in (no error)=w349) -> (queue out=w347:refnum<queue>, error out=w348:errorcluster)  [unwired: 1 in, 1 out]
            n251 = property on="Settings Nav Button" class="Bool (strict)"("DisabledEnum"=T3."Disabled" ("Disabled")) -> ()  [unwired: 2 in, 2 out]
            n252 = property on="Home Nav Button" class="Bool (strict)"("DisabledEnum"=T3."Disabled" ("Disabled")) -> ()  [unwired: 2 in, 2 out]
          }
        }
      }
      event "CtrlNumber": Value Change {
        n253 = event-data() -> ()  [unwired: 1 in, 6 out]
        n254 = local read "CtrlNumberOld"() -> (w353:i32)
        n255 = local read "CtrlNumber"() -> (w352:i32)
        n256 = Not Equal?(x=w353, y=w352) -> (x != y?=w354:bool)
        n257 = case shown="False" w354 {
          frame False {
            n258 = local write "ConfChange"(FALSE ("ConfChange")) -> ()
          }
          frame True {
            n259 = local write "ConfChange"(TRUE ("ConfChange")) -> ()
          }
        }
        n260 = Enqueue Element(queue=w359, element="Numero de controladores", error in (no error)=w357) -> (queue out=w355:refnum<queue>, error out=w356:errorcluster)  [unwired: 1 in, 1 out]
      }
      event "Array CtrlCluster": Value Change {
        n261 = event-data() -> ()  [unwired: 1 in, 6 out]
        n262 = local read "Array CtrlCluster"() -> (w362:T1)
        n263 = local read "CtrlClusterOld"() -> (w363:T1)
        n264 = Not Equal?(x=w363, y=w362) -> (x != y?=w366:bool)
        n265 = case shown="True" w366 {
          frame False {
            n266 = local write "ConfChange"(FALSE ("ConfChange")) -> ()
          }
          frame True {
            n267 = local write "ConfChange"(TRUE ("ConfChange")) -> ()
          }
        }
      }
      event "Read": Value Change {
        n268 = event-data() -> ("NewVal"=w369:bool)  [unwired: 1 in, 5 out]
        n269 = case shown="True" w369 {
          frame False {
            n270 = global write "Variable global de carga.vi" "Conn"(FALSE ("Conn")) -> ()
            n271 = local write "Controllers Load"(T2 [] ("Controllers Load")) -> ()
            n272 = property on="Carga total" class="Bool (strict)"("DisabledEnum"=T3."Enabled" ("Disabled")) -> ()  [unwired: 2 in, 2 out]
            n273 = property on="Settings Nav Button" class="Bool (strict)"("DisabledEnum"=T3."Enabled" ("Disabled")) -> ()  [unwired: 2 in, 2 out]
            n274 = property on="Home Nav Button" class="Bool (strict)"("DisabledEnum"=T3."Enabled" ("Disabled")) -> ()  [unwired: 2 in, 2 out]
          }
          frame True {
            n275 = local write "Loading Text"("" ("Carga texto")) -> ()
            n276 = property on="Carga total" class="Bool (strict)"("DisabledEnum"=T3."Disabled and Grayed Out" ("Disabled")) -> ()  [unwired: 2 in, 2 out]
            n277 = property on="Settings Nav Button" class="Bool (strict)"("DisabledEnum"=T3."Disabled" ("Disabled")) -> ()  [unwired: 2 in, 2 out]
            n278 = property on="Home Nav Button" class="Bool (strict)"("DisabledEnum"=T3."Disabled" ("Disabled")) -> ()  [unwired: 2 in, 2 out]
          }
        }
      }
      event "Secret button": Value Change {
        n279 = event-data() -> ("NewVal"=w381:bool)  [unwired: 1 in, 5 out]
        n280 = case shown="False" w381 {
          frame False {
            n281 = property on="SecretAnimationCtrl" class="DigNum (strict)"("Visible"=FALSE) -> ()  [unwired: 2 in, 2 out]
          }
          frame True {
            n282 = property on="SecretAnimationCtrl" class="DigNum (strict)"("Visible"=TRUE) -> ()  [unwired: 2 in, 2 out]
          }
        }
      }
      event "SecretAnimationCtrl": Value Change {
        n283 = event-data() -> ("NewVal"=w384:i32)  [unwired: 1 in, 5 out]
        n284 = local write "Ring 2"(w384) -> ()
      }
      event "Boton Guardar Cambios": Value Change {
        n285 = event-data() -> ("NewVal"=w385:bool)  [unwired: 1 in, 5 out]
        n286 = case shown="True" w385 {
          tunnel: w389 -> [w391 w396]
          tunnel: w388 -> [w390 w394]
          tunnel: [w390 w393] -> w387
          tunnel: [w391 w392] -> w386
          frame False {
          }
          frame True {
            n287 = Enqueue Element(queue=w396, element="Guardar Cambios", error in (no error)=w394) -> (queue out=w392:refnum<queue>, error out=w393:errorcluster)  [unwired: 1 in, 1 out]
          }
        }
      }
    }
    n288 = case "guard clause" shown="No Error" w258 {
      selector: w258 -> [w259 w261]
      tunnel: w255 -> [w260 w262]
      tunnel: [w260 w264] -> w254
      tunnel: [w259 w263] -> w253
      frame No Error {
        # "No se realiza nada"
      }
      frame Error {
        # "Iniciar el proceso de Shutdown: detener el bucle del consumidor insertando el estado \"Shutdown\" al principio de la cola"
        n289 = Enqueue Element At Opposite End(queue=w262, element="Shutdown", error in (no error)=w261) -> (queue out=w264:refnum<queue>, error out=w263:errorcluster)  [unwired: 1 in, 1 out]
      }
    }
  }
  n290 = Merge Errors(w7, w11) -> (w12:errorcluster)
  n291 = Release Queue(queue=w6, error in (no error)=w12) -> (error out=w10:errorcluster)  [unwired: 1 in, 2 out]
  n292 = call <vilib>:"Simple Error Handler.vi"("error in (no error)"=w10) -> ("error out"=w4:errorcluster)  [unwired: 4 in, 4 out]
  n293 = disable-structure shown="RUN_TIME_ENGINE==True" {
    disable-tunnel: w4 -> [_ _]
    frame condition #0 {
      n294 = Quit LabVIEW() -> ()  [unwired: 1 in]
    }
    frame condition #1 (active) {
    }
  }
  "Ring 2" <- u16 1 ("Ring 2")
